vi "FleaRbRy.vi"() -> ()   [LabVIEW 2013]
doc: "Take a single PixelFly exposure and display the result as an intensity graph.This VI illustrates the basics of taking an exposure with the PixelFly camera. Use Ctrl-H to get help on any of the controls\n\nCopyright 2001, The Cooke Corporation."
uses:
  Shared Libraries/Controls/FileName_Cluster.ctl
  <vilib>/userdefined/High Color/IMAQdx.ctl
  <vilib>/vision/driver/IMAQdx.llb/IMAQdx Acquisition Mode.ctl
  <vilib>/addons/h5labview2/file/H5Fmode.ctl
  Shared Libraries/Controls/FileInfo_Global.vi
  <vilib>/addons/h5labview2/base/lib_path.vi
  <vilib>/addons/h5labview2/base/H5Equery.vi
  <vilib>/addons/h5labview2/base/hid_t.ctl
  <vilib>/addons/h5labview2/dataset/H5Dwrite.llb/H5Dwrite.xnode
  <vilib>/vision/driver/NI_Vision_Acquisition_Software.lvlib
  <vilib>/addons/h5labview2/file/H5F.lvlib
  <vilib>/addons/h5labview2/group/H5G.lvlib
panel:
  in  "Flea Acquire":bool=TRUE
  in  "Interrupt":bool
  out "Status":string="Running..."
  in  "stop":bool
  in  "Tab Control":enum32{"Setup", "Images", "Hardware status"}(tab)
  in  "Do Matlab Analysis":bool
  out "Matlab Command":string
  in  "Save Experimental Parameters to file":enum16{"False", "True"}(ring)
  in  "Flea File Parameters":T1={"Data Root"=path "C:/Data", "Index"=1, "Instrument"="FleaZ"} {"Index" format="%04d"}
  in  "Camera Name":T2="Flea3 FL3-GE-28S4M"
  in  "Experiment":T3(ring)=enum."RbRy"
  in  "Pull Setlist inform string":bool
  in  "Flea Magnification":dbl=1.0
  in  "Flea Image direction":enum16{"XY", "XZ", "ZAxis", "YAxis"}(ring)=enum."ZAxis"
  in  "Flea Imaging technique":enum16{"Absorption", "Fluorescence", "RawImage"}(ring)
  out "Image note":string="Experiment=Sr\nCamera_ID=Flea3_20S4M\nImageType=Raw\nDataType=Absorption\nImageDirection=XZ\nMagnification=6.630000E-1\nWMfreq=4.357345797E+2\nFileNumber=4534\nIndex=27\nIndexedWaves=BlueLaserLockOffset;DipPowX;DipPowX2;DipPowZ;DoppCoolDet;DoppCoolSweep;Nspacers;Pdet;ProbeDet;TOF;TOFaux;WMfreq;Xshim;Yshim;ZshimDC;ZshimVar;bLoadT;bMapT;combWidthF;combWidthI;depumpOn;depumpPow;dopCoolT;freq;holdT;loadT;rMOTbroadDetuningF;rMOTbroadDetuningI;rMOTon;rMOTpow2;rMOTpow3;rMOTpow4;rMOTpow5;rMOTstirDetF;rMOTstirDetI;singleFreqDet;singleFreqStirDet;varWaveP1\nIndexedValues=6.00000000000000E+0;3.00000000000000E+0;3.00000000000000E+0;2.00000000000000E+0;-1.36000000000000E+3;-20.0000000000000E+0;4.00000000000000E+0;4.25000000000000E+0;0.00000000000000E+0;15.0000000000000E-3;8.00000000000000E-3;0.00000000000000E+0;300.000000000000E-3;1.60000000000000E+0;1.65000000000000E+0;1.65000000000000E+0;9.90000000000000E+0;400.000000000000E-6;100.000000000000E-3;1.25000000000000E+0;1.00000000000000E+0;1.00000000000000E+0;75.0000000000000E-3;30.0000000000000E+3;400.000000000000E-3;35.0000000000000E-3;4.77500000000000E+0;4.40000000000000E+0;1.00000000000000E+0;3.00000000000000E+0;7.10000000000000E+0;4.00000000000000E+0;1.15000000000000E+0;4.50000000000000E+0;4.50000000000000E+0;-3.90000000000000E+3;-3.95000000000000E+3;3.50000000000000E+0\n# Current Variables\n#\ndepumpOn = 1.000000E+0\nBBcompT = 4.000000E-1\nBlueLaserLockOffset = 6.000000E+0\nDipPowX = 3.000000E+0\nDipPowX2 = 3.000000E+0\nDipPowXLat = 1.500000E+0\nDipPowZ = 2.000000E+0\nDipPowZ2 = 2.500000E-2\nDipPowZ3 = 2.500000E-2\nDoppCoolDet = -1.360000E+3\nDoppCoolSweep = -2.000000E+1\nHeatingAmp = 1.000000E+0\nMOTPow = 8.000000E+0\nMOTcurrent = -7.500000E+0\nMOTdetuning = -4.504000E+1\nNspacers = 4.000000E+0\nPdet = 4.250000E+0\nPdet2 = 5.000000E-2\nProbeDet = 0.000000E+0\nProbePow = 1.950000E+0\nTOF = 1.500000E-2\nTOFaux = 8.000000E-3\nWMfreq = 0.000000E+0\nXshim = 3.000000E-1\nXshimDC = 6.000000E-1\nYshim = 1.600000E+0\nYshimDC = 1.500000E+0\nZshim = 1.650000E+0\nZshimDC = 1.650000E+0\nZshimVar = 1.650000E+0\nbLoadT = 9.900000E+0\nbMapT = 4.000000E-4\ncombWidthF = 1.000000E-1\ncombWidthI = 1.250000E+0\ncompensation = -3.981000E+0\ndepumpPow = 1.000000E+0\ndopCoolT = 7.500000E-2\ndopCoolT1 = 5.000000E-3\nfreq = 3.000000E+4\nholdT = 4.000000E-1\nloadT = 3.500000E-2\nminus_zman = -7.904000E+0\nplus_zman = -9.792000E+0\nrMOTbroadDetuningF = 4.775000E+0\nrMOTbroadDetuningI = 4.400000E+0\nrMOTcurrF = -2.000000E-1\nrMOTcurrI = -2.000000E-1\nrMOTon = 1.000000E+0\nrMOTpow1 = 7.000000E+0\nrMOTpow2 = 3.000000E+0\nrMOTpow3 = 7.100000E+0\nrMOTpow4 = 4.000000E+0\nrMOTpow5 = 1.150000E+0\nrMOTpow6 = 0.000000E+0\nrMOTstirDetF = 4.500000E+0\nrMOTstirDetI = 4.500000E+0\nsingleFreqDet = -3.900000E+3\nsingleFreqStirDet = -3.950000E+3\nstirWidthF = 1.000000E-1\nstirWidthI = 1.250000E+0\ntEvap0 = 1.000000E-1\ntEvap1 = 2.000000E+0\ntEvap2 = 3.000000E-1\ntau = 6.000000E-1\nvarWaveP1 = 3.500000E+0\nvarWaveP2 = 3.500000E+0\n#\n# Master Staging List\n#Comment\tMarker\tMode\tGroup\tDelay\tX ODT Shuttter\tX ODT AO TTL\tY ODT Shutter\tY ODT AO TTL\tZ ODT Shutter\tZ ODT AO TTL\t707 Shutter\tPB_7\tPB_8\tFreq Switch rMOT\trMOT AO TTL\t\tTrans AO TTL\tProbe AO TTL\tZman AO TTL\tbMOT AO TTL\t60 Hz Trig Gate\tWindow Heater TTL\tPB_18\tPB_19\tPB_20 Trigger Dev3\tPB_21 Trigger Dev2\tPB_22 Trigger Dev1\tPB_23 Trigger Dev0\tStep\t~Atomic Beam Shutter\tGate Valve\tDO0_2\tDO0_3\t~Zman Coils\t~ MOT Coils\t~ Dipole Flea3 Shutter\trMOT Shutter\t+Zeeman Coils\t-Zeeman Coils\tCompensation Coils\tMOT Coils\trMOT AO Power\trMOT Freq Amplitude\trMOT Freq Offset\tAO0_7\tTrans Shutter\tProbe Shutter\tZman Shutter\tbMOT Shutter\tDO1_4\t679 Shutter\t~ Pixis Shutter\t~Abs Flea3 Shutter\tMOT AO Frequency\tMOT AO Power\tProbe AO Power\tProbe AO Frequency\tX Shim Coils\tY Shim Coils\tZ Shim Coils\tZ ODT AO Power\tPIXIS Ext Shutter\tD02_1\tD02_2\tD02_3\tD02_4\tD02_5\tD02_6\tD02_7\tAO2_0\tAO2_1\tD03_0\tD03_1\tD03_2\tD03_3\tD03_4\tD03_5\tD03_6\tD03_7\tAO3_0\tAO3_1\tAO3_2\tVariable Waveplate\t461 Spec Offset\tAO3_5\tAO3_6\tX ODT AO Power\tSRS Freq\tSRS Amp\tSRS Offset\tSRS Func Type\tRedMotDDS\tRedMotDDS_ 0\tRedMotDDS_ 1\tRedMotDDS_ 2\tStirringDDS\tStirringDDS_ 0\tStirringDDS_ 1\tStirringDDS_ 2\r\n\r\nreset\t\tRamp\t1\t.1\t1\t1\t0\t0\t1\t1\t1\t0\t0\t0\t1\t0\t1\t1\t1\t0\t0\t0\t0\t0\t0\t0\t0\t0\t0\t0\t1\t0\t1\t0\t0\t1\t0\tplus_zman\tminus_zman\tcompensation\tMOTcurrent\trMOTpow1\tcombAmplitude(combWidthI)\trMOTdelta(-(rMOTbroadDetuningI +combWidthI/2))\t0\t1\t0\t1\t1\t0\t1\t1\t1\tbMOTdelta(MOTdetuning)\tbMOTpow(0.5)\tProbePow\tPdet2\tXshim\tYshim\tZshim\tODTpowZ(DipPowZ)\t0\t0\t0\t0\t0\t0\t0\t0\t0\t0\t0\t0\t0\t0\t0\t0\t0\t0\trMOTdelta(-(rMOTstirDetI +stirWidthI/2))\tcombAmplitude(stirWidthI)\t0\tvarWaveP1\tBlueLaserLockOffset\tAmp688(depumpPow)\trMOTpow3\tODTpowX(DipPowX)\tfreq\tHeatingAmp\t0\tSine\tDetuning\tsingleFreqDet\t-20\t8\tDetuning\tsingleFreqStirDet\t0\t0\r\nblue MOT load\t\tRamp\t1\tbLoadT\t1\t1\t0\t0\t1\t1\t0\t0\t0\t0\t1\t0\t1\t1\t1\t1\t0\t0\t0\t0\t0\t0\t0\t0\t0\t0\t1\t0\t0\t0\t0\t1\t0\tplus_zman\tminus_zman\tcompensation\tMOTcurrent\trMOTpow1\tcombAmplitude(combWidthI)\trMOTdelta(-(rMOTbroadDetuningI +combWidthI/2))\t0\t1\t0\t1\t1\t0\t1\t1\t1\tbMOTdelta(MOTdetuning)\tbMOTpow(MOTPow)\tProbePow\tPdet2\tXshim\tYshim\tZshim\tODTpowZ(DipPowZ)\t0\tdepumpOn\t0\t0\t0\t0\t0\t0\t0\t0\t0\t0\t0\t0\t0\t0\t0\t0\trMOTdelta(-(rMOTstirDetI +stirWidthI/2))\tcombAmplitude(stirWidthI)\t0\tvarWaveP1\tBlueLaserLockOffset\tAmp688(depumpPow)\trMOTpow3\tODTpowX(DipPowX)\tfreq\tHeatingAmp\t0\tSine\tDetuning\tsingleFreqDet\t-20\t8\tDetuning\tsingleFreqStirDet\t0\t0\r\npretrig\t\tRamp\t1\t6.244e-3\t1\t1\t0\t0\t1\t1\t0\t0\t0\t0\t1\t0\t1\t1\t1\t1\t0\t1\t0\t0\t0\t0\t0\t0\t0\t0\t1\t0\t0\t0\t0\t0\t0\tplus_zman\tminus_zman\tcompensation\tMOTcurrent\trMOTpow1\tcombAmplitude(combWidthI)\trMOTdelta(-(rMOTbroadDetuningI +combWidthI/2))\t0\t1\t0\t1\t1\t0\t1\t0\t0\tbMOTdelta(MOTdetuning)\tbMOTpow(MOTPow)\tProbePow\tPdet2\tXshim\tYshim\tZshim\tODTpowZ(DipPowZ)\t0\tdepumpOn\t0\t0\t0\t0\t0\t0\t0\t0\t0\t0\t0\t0\t0\t0\t0\t0\trMOTdelta(-(rMOTstirDetI +stirWidthI/2))\tcombAmplitude(stirWidthI)\t0\tvarWaveP1\tBlueLaserLockOffset\tAmp688(depumpPow)\trMOTpow3\tODTpowX(DipPowX)\tfreq\tHeatingAmp\t0\tSine\tDetuning\tsingleFreqDet\t-20\t8\tDetuning\tsingleFreqStirDet\t0\t0\r\ndump bMOT\t\tRamp\t1\t0.1\t1\t1\t0\t0\t1\t1\t0\t0\t0\t0\t1\t0\t1\t1\t1\t1\t0\t1\t0\t0\t0\t0\t0\t0\t0\t0\t1\t0\t0\t0\t0\t1\t0\tplus_zman\tminus_zman\tcompensation\tMOTcurrent\trMOTpow1\tcombAmplitude(combWidthI)\trMOTdelta(-(rMOTbroadDetuningI +combWidthI/2))\t0\t1\t0\t1\t1\t0\t1\t1\t1\tbMOTdelta(MOTdetuning)\tbMOTpow(MOTPow)\tProbePow\tPdet2\tXshim\tYshim\tZshim\tODTpowZ(DipPowZ)\t0\tdepumpOn\t0\t0\t0\t0\t0\t0\t0\t0\t0\t0\t0\t0\t0\t0\t0\t0\trMOTdelta(-(rMOTstirDetI +stirWidthI/2))\tcombAmplitude(stirWidthI)\t0\tvarWaveP1\tBlueLaserLockOffset\tAmp688(depumpPow)\trMOTpow3\tODTpowX(DipPowX)\tfreq\tHeatingAmp\t0\tSine\tDetuning\tsingleFreqDet\t-20\t8\tDetuning\tsingleFreqStirDet\t0\t0\r\nCamWaitTime\t\tRamp\t1-rMOTon\t.1\t1\t1\t0\t0\t1\t1\t1\t0\t0\t0\t1\t0\t1\t0\t1\t1\t0\t1\t0\t0\t0\t0\t0\t0\t0\t0\t1\t0\t1\t0\t0\t1\t0\tplus_zman\tminus_zman\tcompensation\tMOTcurrent\trMOTpow1\tcombAmplitude(combWidthI)\trMOTdelta(-(rMOTbroadDetuningI +combWidthI/2))\t0\t1\t1\t1\t1\t0\t1\t1\t1\tbMOTdelta(MOTdetuning)\tbMOTpow(MOTPow)\tProbePow\tPdet2\tXshim\tYshim\tZshim\tODTpowZ(DipPowZ)\t0\t0\t0\t0\t0\t0\t0\t0\t0\t0\t0\t0\t0\t0\t0\t0\t0\t0\trMOTdelta(-(rMOTstirDetI +stirWidthI/2))\tcombAmplitude(stirWidthI)\t0\tvarWaveP1\tBlueLaserLockOffset\tAmp688(depumpPow)\trMOTpow3\tODTpowX(DipPowX)\tfreq\tHeatingAmp\t0\tSine\tDetuning\tsingleFreqDet\t-20\t8\tDetuning\tsingleFreqStirDet\t0\t0\r\nProbeShutOn\t\tRamp\t1-rMOTon\t1120e-6\t1\t1\t0\t0\t1\t1\t1\t0\t0\t0\t1\t0\t0\t0\t0\t1\t0\t1\t0\t0\t0\t0\t0\t0\t0\t0\t1\t0\t1\t0\t0\t1\t1\tplus_zman\tminus_zman\tcompensation\tMOTcurrent\trMOTpow1\tcombAmplitude(combWidthI)\trMOTdelta(-(rMOTbroadDetuningI +combWidthI/2))\t0\t1\t1\t1\t1\t0\t1\t1\t1\tbMOTdelta(MOTdetuning)\tbMOTpow(MOTPow)\tProbePow\tPdet2\tXshim\tYshim\tZshim\tODTpowZ(DipPowZ)\t0\t0\t0\t0\t0\t0\t0\t0\t0\t0\t0\t0\t0\t0\t0\t0\t0\t0\trMOTdelta(-(rMOTstirDetI +stirWidthI/2))\tcombAmplitude(stirWidthI)\t0\tvarWaveP1\tBlueLaserLockOffset\tAmp688(depumpPow)\trMOTpow3\tODTpowX(DipPowX)\tfreq\tHeatingAmp\t0\tSine\tDetuning\tsingleFreqDet\t-20\t8\tDetuning\tsingleFreqStirDet\t0\t0\r\nRepumpShutOff\t\tRamp\t1-rMOTon\t260e-6\t1\t1\t0\t0\t1\t1\t1\t0\t0\t0\t1\t0\t0\t0\t0\t1\t0\t1\t0\t0\t0\t0\t0\t0\t0\t0\t1\t0\t1\t0\t0\t1\t1\tplus_zman\tminus_zman\tcompensation\tMOTcurrent\trMOTpow1\tcombAmplitude(combWidthI)\trMOTdelta(-(rMOTbroadDetuningI +combWidthI/2))\t0\t1\t1\t0\t1\t0\t1\t1\t1\tbMOTdelta(MOTdetuning)\tbMOTpow(MOTPow)\tProbePow\tPdet2\tXshim\tYshim\tZshim\tODTpowZ(DipPowZ)\t0\t0\t0\t0\t0\t0\t0\t0\t0\t0\t0\t0\t0\t0\t0\t0\t0\t0\trMOTdelta(-(rMOTstirDetI +stirWidthI/2))\tcombAmplitude(stirWidthI)\t0\tvarWaveP1\tBlueLaserLockOffset\tAmp688(depumpPow)\trMOTpow3\tODTpowX(DipPowX)\tfreq\tHeatingAmp\t0\tSine\tDetuning\tsingleFreqDet\t-20\t8\tDetuning\tsingleFreqStirDet\t0\t0\r\nMOTShutOff\t\tRamp\t1-rMOTon\t1370e-6\t1\t1\t0\t0\t1\t1\t1\t0\t0\t0\t1\t0\t0\t0\t0\t1\t0\t1\t0\t0\t0\t0\t0\t0\t0\t0\t1\t0\t1\t0\t0\t1\t1\tplus_zman\tminus_zman\tcompensation\tMOTcurrent\trMOTpow1\tcombAmplitude(combWidthI)\trMOTdelta(-(rMOTbroadDetuningI +combWidthI/2))\t0\t1\t1\t0\t0\t0\t1\t1\t1\tbMOTdelta(MOTdetuning)\tbMOTpow(MOTPow)\tProbePow\tPdet2\tXshim\tYshim\tZshim\tODTpowZ(DipPowZ)\t0\t0\t0\t0\t0\t0\t0\t0\t0\t0\t0\t0\t0\t0\t0\t0\t0\t0\trMOTdelta(-(rMOTstirDetI +stirWidthI/2))\tcombAmplitude(stirWidthI)\t0\tvarWaveP1\tBlueLaserLockOffset\tAmp688(depumpPow)\trMOTpow3\tODTpowX(DipPowX)\tfreq\tHeatingAmp\t0\tSine\tDetuning\tsingleFreqDet\t-20\t8\tDetuning\tsingleFreqStirDet\t0\t0\r\nCoil Switch\t\tRamp\trMOTon\t220e-6\t1\t1\t0\t0\t1\t1\t1\t0\t0\t0\t1\t0\t0\t0\t0\t0\t0\t1\t0\t0\t0\t0\t0\t0\t0\t0\t1\t0\t1\t0\t0\t1\t1\tplus_zman\tminus_zman\tcompensation\trMOTcurrI\trMOTpow1\tcombAmplitude(combWidthI)\trMOTdelta(-(rMOTbroadDetuningI +combWidthI/2))\t0\t1\t1\t0\t0\t0\t1\t1\t1\tbMOTdelta(MOTdetuning)\tbMOTpow(0.5)\tProbePow\tPdet2\tXshim\tYshim\tZshim\tODTpowZ(DipPowZ)\t0\t0\t0\t0\t0\t0\t0\t0\t0\t0\t0\t0\t0\t0\t0\t0\t0\t0\trMOTdelta(-(rMOTstirDetI +stirWidthI/2))\tcombAmplitude(stirWidthI)\t0\tvarWaveP1\tBlueLaserLockOffset\tAmp688(depumpPow)\trMOTpow3\tODTpowX(DipPowX)\tfreq\tHeatingAmp\t0\tSine\tDetuning\tsingleFreqDet\t-20\t8\tDetuning\tsingleFreqStirDet\t0\t0\r\n60HzTrigger\t\tHalt\t0\t10u\t1\t1\t0\t0\t1\t1\t1\t0\t0\t0\t1\t0\t0\t0\t0\t0\t1\t1\t0\t0\t0\t0\t0\t0\t0\t0\t1\t0\t1\t0\t0\t1\t1\tplus_zman\tminus_zman\tcompensation\trMOTcurrI\trMOTpow1\tcombAmplitude(combWidthI)\trMOTdelta(-(rMOTbroadDetuningI +combWidthI/2))\t0\t1\t1\t0\t0\t0\t1\t1\t1\tbMOTdelta(MOTdetuning)\tbMOTpow(0.5)\tProbePow\tPdet2\tXshim\tYshim\tZshim\tODTpowZ(DipPowZ)\t0\t0\t0\t0\t0\t0\t0\t0\t0\t0\t0\t0\t0\t0\t0\t0\t0\t0\trMOTdelta(-(rMOTstirDetI +stirWidthI/2))\tcombAmplitude(stirWidthI)\t0\tvarWaveP1\tBlueLaserLockOffset\tAmp688(depumpPow)\trMOTpow3\tODTpowX(DipPowX)\tfreq\tHeatingAmp\t0\tSine\tDetuning\tsingleFreqDet\t-20\t8\tDetuning\tsingleFreqStirDet\t0\t0\r\nCapture Red MOT\t\tRamp\trMOTon\t.175\t1\t1\t0\t0\t1\t0\t1\t0\t0\t0\t1\t0\t0\t0\t0\t0\t0\t1\t0\t0\t0\t0\t0\t0\t0\t0\t1\t0\t1\t0\t0\t1\t1\tplus_zman\tminus_zman\tcompensation\trMOTcurrI\trMOTpow1\tcombAmplitude(combWidthI)\trMOTdelta(-(rMOTbroadDetuningI +combWidthI/2))\t0\t0\t0\t0\t0\t0\t1\t1\t1\tbMOTdelta(MOTdetuning)\tbMOTpow(0.5)\tProbePow\tPdet2\tXshim\tYshim\tZshim\tODTpowZ(DipPowZ)\t0\t0\t0\t0\t0\t0\t0\t0\t0\t0\t0\t0\t0\t0\t0\t0\t0\t0\trMOTdelta(-(rMOTstirDetI +stirWidthI/2))\tcombAmplitude(stirWidthI)\t0\tvarWaveP1\tBlueLaserLockOffset\tAmp688(depumpPow)\trMOTpow3\tODTpowX(DipPowX)\tfreq\tHeatingAmp\t0\tSine\tDetuning\tsingleFreqDet\t-20\t8\tDetuning\tsingleFreqStirDet\t0\t0\r\nRamp Red MOT\t\tRamp\t1\tBBcompT\t1\t1\t0\t0\t1\t0\t1\t0\t0\t0\t1\t0\t0\t0\t0\t0\t0\t1\t0\t0\t0\t0\t0\t0\t10u\t0\t1\t0\t1\t0\t0\t1\t1\tplus_zman\tminus_zman\tcompensation\tLineRamp(f,rMOTcurrI,rMOTcurrF)\tHalfGaussRamp(t,rMOTpow1,rMOTpow2, BBcompT)\tLineRamp(f,combAmplitude(combWidthI),combAmplitude(combWidthF))\tLineRamp(f,rMOTdelta(-(rMOTbroadDetuningI +combWidthI/2)),rMOTdelta(-(rMOTbroadDetuningF +combWidthF/2)))\t0\t0\t0\t0\t0\t0\t1\t0\t1\tbMOTdelta(MOTdetuning)\tbMOTpow(0.5)\tProbePow\tPdet2\tXshim\tYshim\tLineRamp(f,Zshim,ZshimVar)\tODTpowZ(DipPowZ)\t0\t0\t0\t0\t0\t0\t0\t0\t0\t0\t0\t0\t0\t0\t0\t0\t0\t0\tLineRamp(f,rMOTdelta(-(rMOTstirDetI +stirWidthI/2)),rMOTdelta(-(rMOTstirDetF +stirWidthF/2)))\tLineRamp(f,combAmplitude(stirWidthI),combAmplitude(stirWidthF))\t0\tvarWaveP1\tLineRamp(f,BlueLaserLockOffset,Pdet)\tAmp688(depumpPow)\tHalfGaussRamp(t,rMOTpow3,rMOTpow4, BBcompT)\tODTpowX(DipPowX)\tfreq\tHeatingAmp\t0\tSine\tDetuning\tsingleFreqDet\t-20\t8\tDetuning\tsingleFreqStirDet\t0\t0\r\nSF\t\tRamp\t0\t.025\t1\t1\t0\t0\t1\t0\t0\t0\t0\t1\t1\t0\t0\t0\t0\t0\t0\t1\t0\t0\t0\t0\t0\t0\t10u\t0\t1\t0\t0\t0\t0\t1\t1\tplus_zman\tminus_zman\tcompensation\trMOTcurrF\tLineRamp(f,rMOTpow2,rMOTpow2)\tcombAmplitude(combWidthF)\trMOTdelta(-(rMOTbroadDetuningF +combWidthF/2))\t0\t0\t0\t0\t0\t0\t0\t1\t1\tbMOTdelta(MOTdetuning)\tbMOTpow(0.5)\tProbePow\tPdet2\tXshim\tYshim\tZshimVar\tODTpowZ(DipPowZ)\t0\t0\t0\t0\t0\t0\t0\t0\t0\t0\t0\t0\t0\t0\t0\t0\t0\t0\trMOTdelta(-(rMOTstirDetI +stirWidthF/2))\tcombAmplitude(stirWidthF)\t0\tvarWaveP1\tPdet\tAmp688(depumpPow)\tLineRamp(f,rMOTpow4,rMOTpow4)\tODTpowX(DipPowX)\tfreq\tHeatingAmp\t0\tSine\tDetuning\tsingleFreqDet\t-20\t8\tDetuning\tsingleFreqStirDet\t0\t0\r\nload1\t\tRamp\t0\tloadT\t1\t1\t0\t0\t1\t0\t0\t0\t0\t1\t1\t0\t0\t1\t0\t0\t0\t1\t0\t0\t0\t0\t0\t0\t0\t0\t1\t0\t0\t0\t0\t1\t1\tplus_zman\tminus_zman\tcompensation\trMOTcurrF\trMOTpow3\tcombAmplitude(combWidthF)\trMOTdelta(-(rMOTbroadDetuningF +combWidthF/2))\t0\t0\t0\t0\t0\t0\t0\t1\t1\tbMOTdelta(MOTdetuning)\tbMOTpow(0.5)\tProbePow\tPdet2\tXshim\tYshim\tZshimVar\tODTpowZ(DipPowZ)\t0\t0\t0\t0\t0\t0\t0\t0\t0\t0\t0\t0\t0\t0\t0\t0\t0\t0\trMOTdelta(-(rMOTstirDetI +stirWidthF/2))\tcombAmplitude(stirWidthF)\t0\tvarWaveP1\tPdet\tAmp688(depumpPow)\trMOTpow3\tODTpowX(DipPowX)\tfreq\tHeatingAmp\t0\tSine\tDetuning\tsingleFreqDet\t-20\t8\tDetuning\tsingleFreqStirDet\t0\t0\r\nload2\t\tRamp\t0\t.05\t1\t1\t0\t0\t1\t0\t0\t0\t0\t1\t1\t0\t0\t1\t0\t0\t0\t1\t0\t0\t0\t0\t0\t0\t0\t0\t1\t0\t0\t0\t0\t1\t1\tplus_zman\tminus_zman\tcompensation\trMOTcurrF\trMOTpow3\tcombAmplitude(combWidthF)\trMOTdelta(-(rMOTbroadDetuningF +combWidthF/2))\t0\t0\t0\t0\t0\t0\t0\t1\t1\tbMOTdelta(MOTdetuning)\tbMOTpow(0.5)\tProbePow\tPdet2\tXshim\tYshim\tZshimVar\tODTpowZ(DipPowZ)\t0\t0\t0\t0\t0\t0\t0\t0\t0\t0\t0\t0\t0\t0\t0\t0\t0\t0\trMOTdelta(-(rMOTstirDetI +stirWidthF/2))\tcombAmplitude(stirWidthF)\t0\tvarWaveP1\tPdet\tAmp688(depumpPow)\trMOTpow3\tODTpowX(DipPowX)\tfreq\tHeatingAmp\t0\tSine\tDetuning\tsingleFreqDet\t-20\t8\tDetuning\tsingleFreqStirDet\t0\t0\r\ndrop Red MOT\t\tRamp\t0\t.05\t1\t1\t0\t0\t1\t0\t0\t0\t0\t1\t0\t0\t0\t1\t0\t0\t0\t1\t0\t0\t0\t0\t0\t0\t10u\t0\t1\t0\t0\t0\t1\t1\t0\tplus_zman\tminus_zman\tcompensation\trMOTcurrF\trMOTpow3\tcombAmplitude(combWidthF)\trMOTdelta(-(rMOTbroadDetuningF +combWidthF/2))\t0\t0\t0\t0\t0\t0\t0\t1\t1\tbMOTdelta(MOTdetuning)\tbMOTpow(0.5)\tProbePow\tPdet2\tLineRamp(f,Xshim,XshimDC)\tLineRamp(f,Yshim,YshimDC)\tLineRamp(f,ZshimVar,ZshimDC)\tODTpowZ(DipPowZ)\t0\t0\t0\t0\t0\t0\t0\t0\t0\t0\t0\t0\t0\t0\t0\t0\t0\t0\trMOTdelta(-(rMOTstirDetI +stirWidthF/2))\tcombAmplitude(stirWidthF)\t0\tvarWaveP1\tPdet\tAmp688(depumpPow)\trMOTpow3\tODTpowX(DipPowX)\tfreq\tHeatingAmp\t0\tSine\tDetuning\tsingleFreqDet\t-20\t8\tDetuning\tsingleFreqStirDet\t0\t0\r\nramp Trap\t\tRamp\t0\t.05\t1\t1\t0\t0\t1\t0\t0\t0\t0\t1\t0\t0\t0\t1\t0\t0\t0\t1\t0\t0\t0\t0\t0\t0\t10u\t0\t1\t0\t0\t0\t1\t1\t0\tplus_zman\tminus_zman\tcompensation\trMOTcurrF\trMOTpow3\tcombAmplitude(combWidthF)\trMOTdelta(-(rMOTbroadDetuningF +combWidthF/2))\t0\t0\t0\t0\t0\t0\t0\t1\t1\tbMOTdelta(MOTdetuning)\tbMOTpow(0.5)\tProbePow\tPdet2\tXshimDC\tYshimDC\tZshimDC\tODTpowZ(DipPowZ)\t0\t0\t0\t0\t0\t0\t0\t0\t0\t0\t0\t0\t0\t0\t0\t0\t0\t0\trMOTdelta(-(rMOTstirDetI +stirWidthF/2))\tcombAmplitude(stirWidthF)\t0\tvarWaveP1\tPdet\tAmp688(depumpPow)\trMOTpow3\tSinRamp(t,(ODTpowX(DipPowX)+ODTpowX(DipPowX2))/2,(ODTpowX(DipPowX2)-ODTpowX(DipPowX))/2,10,3*pi/2)\tfreq\tHeatingAmp\t0\tSine\tDetuning\tsingleFreqDet\t-20\t8\tDetuning\tsingleFreqStirDet\t0\t0\r\nhold\t\tRamp\t0\t5\t1\t1\t0\t0\t1\t0\t0\t0\t0\t1\t0\t0\t0\t1\t0\t0\t0\t1\t0\t0\t0\t0\t0\t0\t0\t0\t1\t0\t0\t0\t1\t1\t1\tplus_zman\tminus_zman\tcompensation\trMOTcurrF\trMOTpow4\tcombAmplitude(combWidthF)\trMOTdelta(-(rMOTbroadDetuningF +combWidthF/2))\t0\t0\t0\t0\t0\t0\t0\t1\t1\tbMOTdelta(MOTdetuning)\tbMOTpow(0.5)\tProbePow\tPdet2\tXshimDC\tYshimDC\tZshimDC\tODTpowZ(DipPowZ)\t0\t0\t0\t0\t0\t0\t0\t0\t0\t0\t0\t0\t0\t0\t0\t0\t0\t0\trMOTdelta(-(rMOTstirDetI +stirWidthF/2))\tcombAmplitude(stirWidthF)\t0\tvarWaveP1\tPdet\tAmp688(depumpPow)\trMOTpow4\tODTpowX(DipPowX2)\tfreq\tHeatingAmp\t0\tSine\tDetuning\tDoppCoolDet\t-20\t8\tDetuning\tsingleFreqStirDet\t0\t0\r\nDoppler Cool1\t\tRamp\t0\tdopCoolT\t1\t1\t0\t0\t1\t0\t0\t0\t0\t1\t1\t0\t0\t1\t0\t0\t0\t1\t0\t0\t0\t0\t0\t0\t10u\t0\t1\t0\t0\t0\t1\t1\t1\tplus_zman\tminus_zman\tcompensation\trMOTcurrF\tLineRamp(f,rMOTpow4,1.15)\tcombAmplitude(combWidthF)\trMOTdelta(-(rMOTbroadDetuningF +combWidthF/2))\t0\t0\t0\t0\t0\t0\t0\t1\t1\tbMOTdelta(MOTdetuning)\tbMOTpow(0.5)\tProbePow\tPdet2\tXshimDC\tYshimDC\tZshimDC\tODTpowZ(DipPowZ)\t0\t0\t0\t0\t0\t0\t0\t0\t0\t0\t0\t0\t0\t0\t0\t0\t0\t0\trMOTdelta(-(rMOTstirDetI +stirWidthF/2))\tcombAmplitude(stirWidthF)\t0\tvarWaveP1\tPdet\tAmp688(depumpPow)\tLineRamp(f,rMOTpow4,1.15)\tODTpowX(DipPowX2)\tfreq\tHeatingAmp\t0\tSine\tDetuning\tDoppCoolDet\t-20\t8\tDetuning\tsingleFreqStirDet\t0\t0\r\nDoppler Cool2\t\tRamp\t0\tdopCoolT\t1\t1\t0\t0\t1\t0\t0\t0\t0\t1\t1\t0\t0\t1\t0\t0\t0\t1\t0\t0\t0\t0\t0\t0\t10u\t0\t1\t0\t0\t0\t1\t1\t1\tplus_zman\tminus_zman\tcompensation\trMOTcurrF\trMOTpow4\tcombAmplitude(combWidthF)\trMOTdelta(-(rMOTbroadDetuningF +combWidthF/2))\t0\t0\t0\t0\t0\t0\t0\t1\t1\tbMOTdelta(MOTdetuning)\tbMOTpow(0.5)\tProbePow\tPdet2\tXshimDC\tYshimDC\tZshimDC\tODTpowZ(DipPowZ)\t0\t0\t0\t0\t0\t0\t0\t0\t0\t0\t0\t0\t0\t0\t0\t0\t0\t0\trMOTdelta(-(rMOTstirDetI +stirWidthF/2))\tcombAmplitude(stirWidthF)\t0\tvarWaveP1\tPdet\tAmp688(depumpPow)\trMOTpow4\tODTpowX(DipPowX2)\tfreq\tHeatingAmp\t0\tSine\tRamp\tDoppCoolDet\tDoppCoolDet-DoppCoolSweep\tdopCoolT*1000\tDetuning\tsingleFreqStirDet\t0\t0\r\nDoppler Cool3\t\tRamp\t0\tdopCoolT\t1\t1\t0\t0\t1\t0\t0\t0\t0\t1\t1\t0\t0\t1\t0\t0\t0\t1\t0\t0\t0\t0\t0\t0\t10u\t0\t1\t0\t0\t0\t1\t1\t1\tplus_zman\tminus_zman\tcompensation\trMOTcurrF\tLineRamp(f,rMOTpow4,rMOTpow5)\tcombAmplitude(combWidthF)\trMOTdelta(-(rMOTbroadDetuningF +combWidthF/2))\t0\t0\t0\t0\t0\t0\t0\t1\t1\tbMOTdelta(MOTdetuning)\tbMOTpow(0.5)\tProbePow\tPdet2\tXshimDC\tYshimDC\tZshimDC\tODTpowZ(DipPowZ)\t0\t0\t0\t0\t0\t0\t0\t0\t0\t0\t0\t0\t0\t0\t0\t0\t0\t0\trMOTdelta(-(rMOTstirDetI +stirWidthF/2))\tcombAmplitude(stirWidthF)\t0\tvarWaveP1\tPdet\tAmp688(depumpPow)\tLineRamp(f,rMOTpow4,rMOTpow5)\tODTpowX(DipPowX2)\tfreq\tHeatingAmp\t0\tSine\tDetuning\tDoppCoolDet-DoppCoolSweep\tDoppCoolDet-DoppCoolSweep\tdopCoolT*1000\tDetuning\tsingleFreqStirDet\t0\t0\r\nhold\t\tRamp\t0\tholdT\t1\t1\t0\t0\t1\t0\t0\t0\t0\t1\t0\t0\t0\t1\t0\t0\t0\t1\t1\t0\t0\t0\t0\t0\t0\t0\t1\t0\t0\t0\t1\t1\t0\tplus_zman\tminus_zman\tcompensation\trMOTcurrF\trMOTpow4\tcombAmplitude(combWidthF)\trMOTdelta(-(rMOTbroadDetuningF +combWidthF/2))\t0\t1\t0\t0\t0\t0\t0\t1\t1\tbMOTdelta(MOTdetuning)\tbMOTpow(0.5)\tProbePow\tPdet2\tXshim\tYshim\tZshimVar\tODTpowZ(DipPowZ)\t0\t0\t0\t0\t0\t0\t0\t0\t0\t0\t0\t0\t0\t0\t0\t0\t0\t0\trMOTdelta(-(rMOTstirDetI +stirWidthF/2))\tcombAmplitude(stirWidthF)\t0\tvarWaveP1\tPdet\tAmp688(depumpPow)\trMOTpow4\tODTpowX(DipPowX2)\tfreq\tHeatingAmp\t0\tSine\tDetuning\tDoppCoolDet-DoppCoolSweep\tDoppCoolDet-DoppCoolSweep\tdopCoolT*1000\tDetuning\tsingleFreqStirDet\t0\t0\r\ndrop HTrap\t\tRamp\t0\t.03\t1\t1\t0\t0\t1\t0\t1\t0\t0\t1\t0\t0\t0\t1\t0\t0\t0\t1\t0\t0\t0\t0\t0\t0\t0\t0\t1\t0\t0\t0\t0\t1\t0\tplus_zman\tminus_zman\tcompensation\trMOTcurrF\trMOTpow3\tcombAmplitude(combWidthF)\trMOTdelta(-(rMOTbroadDetuningF +combWidthF/2))\t0\t1\t0\t0\t0\t0\t1\t1\t1\tbMOTdelta(MOTdetuning)\tbMOTpow(0.5)\tProbePow\tPdet2\tXshim\tYshim\tZshimVar\tODTpowZ(DipPowZ)\t0\t0\t0\t0\t0\t0\t0\t0\t0\t0\t0\t0\t0\t0\t0\t0\t0\t0\trMOTdelta(-(rMOTstirDetI +stirWidthF/2))\tcombAmplitude(stirWidthF)\t0\tvarWaveP1\tPdet\tAmp688(depumpPow)\trMOTpow3\tODTpowX(DipPowX)\tfreq\tHeatingAmp\t0\tSine\tDetuning\tsingleFreqDet\tDoppCoolDet-DoppCoolSweep\tdopCoolT*1000\tDetuning\tsingleFreqStirDet\t0\t0\r\nmodulate\t\tRamp\t0\t3m\t1\t1\t0\t0\t1\t0\t1\t0\t0\t1\t0\t0\t0\t1\t0\t0\t0\t1\t0\t0\t0\t0\t0\t0\t0\t0\t1\t0\t0\t0\t0\t1\t0\tplus_zman\tminus_zman\tcompensation\trMOTcurrF\trMOTpow3\tcombAmplitude(combWidthF)\trMOTdelta(-(rMOTbroadDetuningF +combWidthF/2))\t0\t1\t0\t0\t0\t0\t1\t1\t1\tbMOTdelta(MOTdetuning)\tbMOTpow(0.5)\tProbePow\tPdet2\tXshim\tYshim\tZshimVar\tODTpowZ(DipPowZ)\t0\t0\t0\t0\t0\t0\t0\t0\t0\t0\t0\t0\t0\t0\t0\t0\t0\t0\trMOTdelta(-(rMOTstirDetI +stirWidthF/2))\tcombAmplitude(stirWidthF)\t0\tvarWaveP1\tPdet\tAmp688(depumpPow)\trMOTpow3\tODTpowX(DipPowX)\tfreq\tHeatingAmp\t0\tSine\tDetuning\tsingleFreqDet\tDoppCoolDet-DoppCoolSweep\tdopCoolT*1000\tDetuning\tsingleFreqStirDet\t0\t0\r\nEvaporation\t\tRamp\t0\ttEvap1\t1\t1\t0\t0\t1\t0\t1\t0\t0\t1\t0\t0\t0\t1\t0\t0\t0\t1\t0\t0\t0\t0\t0\t0\t1m\t0\t1\t0\t0\t0\t0\t1\t0\tplus_zman\tminus_zman\tcompensation\trMOTcurrF\trMOTpow3\tcombAmplitude(combWidthF)\trMOTdelta(-(rMOTbroadDetuningF +combWidthF/2))\t0\t1\t0\t0\t0\t0\t1\t1\t1\tbMOTdelta(MOTdetuning)\tbMOTpow(0.5)\tProbePow\tPdet2\tXshim\tYshim\tZshimVar\tODTpowZ(DipPowZ)\t0\t0\t0\t0\t0\t0\t0\t0\t0\t0\t0\t0\t0\t0\t0\t0\t0\t0\trMOTdelta(-(rMOTstirDetI +stirWidthF/2))\tcombAmplitude(stirWidthF)\t0\tvarWaveP1\tPdet\tAmp688(depumpPow)\trMOTpow3\tExpRamp2(t,0,ODTpowX(DipPowX),ODTpowX(DipPowX2),tau)\tfreq\tHeatingAmp\t0\tSine\tDetuning\tsingleFreqDet\tDoppCoolDet-DoppCoolSweep\tdopCoolT*1000\tDetuning\tsingleFreqStirDet\t0\t0\r\ndrop\t\tRamp\t0\t.01\t1\t1\t0\t0\t1\t0\t1\t0\t0\t1\t0\t0\t0\t1\t0\t0\t0\t1\t0\t0\t0\t0\t0\t0\t0\t0\t1\t0\t0\t0\t0\t1\t0\tplus_zman\tminus_zman\tcompensation\trMOTcurrF\trMOTpow3\tcombAmplitude(combWidthF)\trMOTdelta(-(rMOTbroadDetuningF +combWidthF/2))\t0\t1\t0\t0\t0\t0\t1\t1\t1\tbMOTdelta(MOTdetuning)\tbMOTpow(0.5)\tProbePow\tPdet2\tXshim\tYshim\tZshimVar\tODTpowZ(DipPowZ)\t0\t0\t0\t0\t0\t0\t0\t0\t0\t0\t0\t0\t0\t0\t0\t0\t0\t0\trMOTdelta(-(rMOTstirDetI +stirWidthF/2))\tcombAmplitude(stirWidthF)\t0\tvarWaveP2\tPdet\tAmp688(depumpPow)\trMOTpow3\tODTpowX(DipPowXLat)\tfreq\tHeatingAmp\t0\tSine\tDetuning\tsingleFreqDet\tDoppCoolDet-DoppCoolSweep\tdopCoolT*1000\tDetuning\tsingleFreqStirDet\t0\t0\r\nband map\t\tRamp\t0\tbMapT\t1\t1\t0\t0\t1\t0\t1\t0\t0\t1\t0\t0\t0\t1\t0\t0\t0\t1\t0\t0\t0\t0\t0\t0\t2u\t0\t1\t0\t0\t0\t0\t1\t0\tplus_zman\tminus_zman\tcompensation\trMOTcurrF\trMOTpow3\tcombAmplitude(combWidthF)\trMOTdelta(-(rMOTbroadDetuningF +combWidthF/2))\t0\t1\t0\t0\t0\t0\t1\t1\t1\tbMOTdelta(MOTdetuning)\tbMOTpow(0.5)\tProbePow\tPdet2\tXshim\tYshim\tZshimVar\tLineRamp(f,ODTpowZ(DipPowZ),ODTpowZ(-0.2))\t0\t0\t0\t0\t0\t0\t0\t0\t0\t0\t0\t0\t0\t0\t0\t0\t0\t0\trMOTdelta(-(rMOTstirDetI +stirWidthF/2))\tcombAmplitude(stirWidthF)\t0\tvarWaveP2\tPdet\tAmp688(depumpPow)\trMOTpow3\tLineRamp(f,ODTpowX(DipPowX),0)\tfreq\tHeatingAmp\t0\tSine\tDetuning\tsingleFreqDet\tDoppCoolDet-DoppCoolSweep\tdopCoolT*1000\tDetuning\tsingleFreqStirDet\t0\t0\r\nband map delay\t\tRamp\t0\t10u\t1\t1\t0\t0\t1\t0\t1\t0\t0\t1\t0\t0\t0\t1\t0\t0\t0\t1\t0\t0\t0\t0\t0\t0\t0\t0\t1\t0\t0\t0\t0\t1\t0\tplus_zman\tminus_zman\tcompensation\trMOTcurrF\trMOTpow3\tcombAmplitude(combWidthF)\trMOTdelta(-(rMOTbroadDetuningF +combWidthF/2))\t0\t1\t0\t0\t0\t0\t1\t1\t1\tbMOTdelta(MOTdetuning)\tbMOTpow(0.5)\tProbePow\tPdet2\tXshim\tYshim\tZshimVar\tODTpowZ(DipPowZ)\t0\t0\t0\t0\t0\t0\t0\t0\t0\t0\t0\t0\t0\t0\t0\t0\t0\t0\trMOTdelta(-(rMOTstirDetI +stirWidthF/2))\tcombAmplitude(stirWidthF)\t0\tvarWaveP2\tPdet\tAmp688(depumpPow)\trMOTpow3\tODTpowX(DipPowXLat)\tfreq\tHeatingAmp\t0\tSine\tDetuning\tsingleFreqDet\tDoppCoolDet-DoppCoolSweep\tdopCoolT*1000\tDetuning\tsingleFreqStirDet\t0\t0\r\nTOF\t\tRamp\t0\tTOFaux\t0\t0\t0\t0\t0\t0\t1\t0\t0\t0\t0\t0\t0\t0\t0\t0\t0\t1\t0\t0\t0\t0\t0\t0\t0\t0\t1\t0\t0\t0\t1\t1\t0\tplus_zman\tminus_zman\tcompensation\trMOTcurrF\trMOTpow3\tcombAmplitude(combWidthF)\trMOTdelta(-(rMOTbroadDetuningF +combWidthF/2))\t0\t1\t1\t0\t0\t0\t1\t1\t1\tbMOTdelta(MOTdetuning)\tbMOTpow(0.5)\tProbePow\tPdet\tXshim\tYshim\tZshimVar\tODTpowZ(DipPowZ)\t1\t0\t0\t0\t0\t0\t0\t0\t0\t0\t0\t0\t0\t0\t0\t0\t0\t0\trMOTdelta(-(rMOTstirDetI +stirWidthF/2))\tcombAmplitude(stirWidthF)\t0\tvarWaveP2\tPdet\tAmp688(depumpPow)\trMOTpow3\tODTpowX(DipPowX2)\tfreq\tHeatingAmp\t0\tSine\tDetuning\tsingleFreqDet\tDoppCoolDet-DoppCoolSweep\tdopCoolT*1000\tDetuning\tsingleFreqStirDet\t0\t0\r\nTOF\t\tRamp\trMOTon\t.005\t0\t0\t0\t0\t0\t0\t1\t0\t0\t0\t0\t0\t0\t0\t0\t0\t0\t1\t0\t0\t0\t0\t0\t0\t0\t0\t1\t0\t0\t0\t1\t1\t0\tplus_zman\tminus_zman\tcompensation\trMOTcurrF\trMOTpow3\tcombAmplitude(combWidthF)\trMOTdelta(-(rMOTbroadDetuningF +combWidthF/2))\t0\t1\t1\t0\t0\t0\t1\t1\t1\tbMOTdelta(MOTdetuning)\tbMOTpow(0.5)\tProbePow\tPdet\tXshim\tYshim\tZshimVar\tODTpowZ(DipPowZ)\t1\t0\t0\t0\t0\t0\t0\t0\t0\t0\t0\t0\t0\t0\t0\t0\t0\t0\trMOTdelta(-(rMOTstirDetI +stirWidthF/2))\tcombAmplitude(stirWidthF)\t0\tvarWaveP2\tPdet\tAmp688(depumpPow)\trMOTpow3\tODTpowX(DipPowX2)\tfreq\tHeatingAmp\t0\tSine\tDetuning\tsingleFreqDet\tDoppCoolDet-DoppCoolSweep\tdopCoolT*1000\tDetuning\tsingleFreqStirDet\t0\t0\r\nTOF\t\tRamp\t1-rMOTon\t.001\t0\t0\t0\t0\t0\t0\t1\t0\t0\t0\t0\t0\t0\t0\t0\t0\t0\t1\t0\t0\t0\t0\t0\t0\t0\t0\t1\t0\t0\t0\t1\t1\t0\tplus_zman\tminus_zman\tcompensation\trMOTcurrF\trMOTpow3\tcombAmplitude(combWidthF)\trMOTdelta(-(rMOTbroadDetuningF +combWidthF/2))\t0\t1\t1\t0\t0\t0\t1\t1\t1\tbMOTdelta(MOTdetuning)\tbMOTpow(0.5)\tProbePow\tPdet\tXshim\tYshim\tZshimVar\tODTpowZ(DipPowZ)\t1\t0\t0\t0\t0\t0\t0\t0\t0\t0\t0\t0\t0\t0\t0\t0\t0\t0\trMOTdelta(-(rMOTstirDetI +stirWidthF/2))\tcombAmplitude(stirWidthF)\t0\tvarWaveP2\tPdet\tAmp688(depumpPow)\trMOTpow3\tODTpowX(DipPowX2)\tfreq\tHeatingAmp\t0\tSine\tDetuning\tsingleFreqDet\tDoppCoolDet-DoppCoolSweep\tdopCoolT*1000\tDetuning\tsingleFreqStirDet\t0\t0\r\narm FLEA\t\tRamp\t1\t.000044\t0\t0\t0\t0\t0\t0\t1\t0\t0\t0\t0\t0\t0\t0\t0\t0\t0\t0\t0\t0\t0\t0\t0\t0\t0\t0\t1\t0\t0\t0\t1\t0\t0\tplus_zman\tminus_zman\tcompensation\trMOTcurrF\trMOTpow3\tcombAmplitude(combWidthF)\trMOTdelta(-(rMOTbroadDetuningF +combWidthF/2))\t0\t1\t1\t0\t0\t0\t1\t1\t0\tbMOTdelta(MOTdetuning)\tbMOTpow(0.5)\tProbePow\tPdet\tXshim\tYshim\tZshimVar\tODTpowZ(0)\t1\t0\t0\t0\t0\t0\t0\t0\t0\t0\t0\t0\t0\t0\t0\t0\t0\t0\trMOTdelta(-(rMOTstirDetI +stirWidthF/2))\tcombAmplitude(stirWidthF)\t0\tvarWaveP2\tPdet\tAmp688(depumpPow)\trMOTpow3\tODTpowX(DipPowX)\tfreq\tHeatingAmp\t0\tSine\tDetuning\tsingleFreqDet\tDoppCoolDet-DoppCoolSweep\tdopCoolT*1000\tDetuning\tsingleFreqStirDet\t0\t0\r\natom img\t\tRamp\t1\t10e-6\t0\t0\t0\t0\t0\t0\t1\t0\t0\t0\t0\t0\t0\t1\t0\t0\t0\t0\t0\t0\t0\t0\t0\t0\t0\t0\t1\t0\t0\t0\t1\t0\t0\tplus_zman\tminus_zman\tcompensation\trMOTcurrF\trMOTpow3\tcombAmplitude(combWidthF)\trMOTdelta(-(rMOTbroadDetuningF +combWidthF/2))\t0\t1\t1\t0\t0\t0\t1\t0\t0\tbMOTdelta(MOTdetuning)\tbMOTpow(0.5)\tProbePow\tPdet\tXshim\tYshim\tZshimVar\tODTpowZ(0)\t1\t0\t0\t0\t0\t0\t0\t0\t0\t0\t0\t0\t0\t0\t0\t0\t0\t0\trMOTdelta(-(rMOTstirDetI +stirWidthF/2))\tcombAmplitude(stirWidthF)\t0\tvarWaveP2\tPdet\tAmp688(depumpPow)\trMOTpow3\tODTpowX(DipPowX)\tfreq\tHeatingAmp\t0\tSine\tDetuning\tsingleFreqDet\tDoppCoolDet-DoppCoolSweep\tdopCoolT*1000\tDetuning\tsingleFreqStirDet\t0\t0\r\natom img\t\tRamp\t0\t2.8e-3\t0\t0\t0\t0\t0\t0\t1\t0\t0\t1\t0\t0\t0\t0\t0\t0\t0\t0\t0\t0\t0\t0\t0\t0\t0\t0\t1\t0\t0\t0\t1\t1\t0\tplus_zman\tminus_zman\tcompensation\trMOTcurrF\trMOTpow3\tcombAmplitude(combWidthF)\trMOTdelta(-(rMOTbroadDetuningF +combWidthF/2))\t0\t1\t1\t0\t0\t0\t1\t1\t1\tbMOTdelta(MOTdetuning)\tbMOTpow(0.5)\tProbePow\tPdet\tXshim\tYshim\tZshimVar\tODTpowZ(DipPowZ)\t1\t0\t0\t0\t0\t0\t0\t0\t0\t0\t0\t0\t0\t0\t0\t0\t0\t0\trMOTdelta(-(rMOTstirDetI +stirWidthF/2))\tcombAmplitude(stirWidthF)\t0\tvarWaveP2\tPdet\tAmp688(depumpPow)\trMOTpow3\tODTpowX(DipPowX)\tfreq\tHeatingAmp\t0\tSine\tDetuning\tsingleFreqDet\tDoppCoolDet-DoppCoolSweep\tdopCoolT*1000\tDetuning\tsingleFreqStirDet\t0\t0\r\ntransmit img\t\tRamp\t1\t.300\t0\t0\t0\t0\t0\t0\t1\t0\t0\t1\t0\t0\t0\t0\t0\t0\t0\t0\t0\t0\t0\t0\t0\t0\t0\t0\t1\t0\t0\t0\t1\t1\t0\tplus_zman\tminus_zman\tcompensation\trMOTcurrF\trMOTpow3\tcombAmplitude(combWidthF)\trMOTdelta(-(rMOTbroadDetuningF +combWidthF/2))\t0\t1\t1\t0\t0\t0\t1\t1\t1\tbMOTdelta(MOTdetuning)\tbMOTpow(0.5)\tProbePow\tPdet\tXshim\tYshim\tZshimVar\tODTpowZ(DipPowZ)\t1\t0\t0\t0\t0\t0\t0\t0\t0\t0\t0\t0\t0\t0\t0\t0\t0\t0\trMOTdelta(-(rMOTstirDetI +stirWidthF/2))\tcombAmplitude(stirWidthF)\t0\tvarWaveP2\tPdet\tAmp688(depumpPow)\trMOTpow3\tODTpowX(DipPowX)\tfreq\tHeatingAmp\t0\tSine\tDetuning\tsingleFreqDet\tDoppCoolDet-DoppCoolSweep\tdopCoolT*1000\tDetuning\tsingleFreqStirDet\t0\t0\r\narm PIXIS\t\tRamp\t1\t.007\t1\t1\t0\t0\t0\t1\t1\t0\t0\t1\t1\t0\t0\t0\t1\t1\t0\t0\t0\t0\t0\t0\t0\t0\t0\t0\t1\t0\t0\t0\t1\t1\t0\tplus_zman\tminus_zman\tcompensation\trMOTcurrF\trMOTpow1\tcombAmplitude(combWidthF)\trMOTdelta(-(rMOTbroadDetuningF +combWidthF/2))\t0\t1\t1\t0\t0\t0\t1\t1\t1\tbMOTdelta(MOTdetuning)\tbMOTpow(0.5)\tProbePow\tPdet\tXshim\tYshim\tZshimVar\tODTpowZ(DipPowZ)\t1\t0\t0\t0\t0\t0\t0\t0\t0\t0\t0\t0\t0\t0\t0\t0\t0\t0\trMOTdelta(-(rMOTstirDetI +stirWidthF/2))\tcombAmplitude(stirWidthF)\t0\tvarWaveP2\tPdet\tAmp688(depumpPow)\trMOTpow1\tODTpowX(DipPowX)\tfreq\tHeatingAmp\t0\tSine\tDetuning\tsingleFreqDet\tDoppCoolDet-DoppCoolSweep\tdopCoolT*1000\tDetuning\tsingleFreqStirDet\t0\t0\r\narm FLEA\t\tRamp\t1\t44e-6\t1\t1\t0\t0\t0\t1\t1\t0\t0\t1\t1\t0\t0\t0\t1\t1\t0\t0\t0\t0\t0\t0\t0\t0\t0\t0\t1\t0\t0\t0\t1\t0\t0\tplus_zman\tminus_zman\tcompensation\trMOTcurrF\trMOTpow1\tcombAmplitude(combWidthF)\trMOTdelta(-(rMOTbroadDetuningF +combWidthF/2))\t0\t1\t1\t0\t0\t0\t1\t1\t0\tbMOTdelta(MOTdetuning)\tbMOTpow(0.5)\tProbePow\tPdet\tXshim\tYshim\tZshimVar\tODTpowZ(DipPowZ)\t1\t0\t0\t0\t0\t0\t0\t0\t0\t0\t0\t0\t0\t0\t0\t0\t0\t0\trMOTdelta(-(rMOTstirDetI +stirWidthF/2))\tcombAmplitude(stirWidthF)\t0\tvarWaveP2\tPdet\tAmp688(depumpPow)\trMOTpow1\tODTpowX(DipPowX)\tfreq\tHeatingAmp\t0\tSine\tDetuning\tsingleFreqDet\tDoppCoolDet-DoppCoolSweep\tdopCoolT*1000\tDetuning\tsingleFreqStirDet\t0\t0\r\nprobe img\t\tRamp\t1\t10e-6\t1\t1\t0\t0\t0\t1\t1\t0\t0\t1\t1\t0\t0\t1\t1\t1\t0\t0\t0\t0\t0\t0\t0\t0\t0\t0\t1\t0\t0\t0\t1\t0\t0\tplus_zman\tminus_zman\tcompensation\trMOTcurrF\trMOTpow1\tcombAmplitude(combWidthF)\trMOTdelta(-(rMOTbroadDetuningF +combWidthF/2))\t0\t1\t1\t0\t0\t0\t1\t0\t0\tbMOTdelta(MOTdetuning)\tbMOTpow(0.5)\tProbePow\tPdet\tXshim\tYshim\tZshimVar\tODTpowZ(DipPowZ)\t1\t0\t0\t0\t0\t0\t0\t0\t0\t0\t0\t0\t0\t0\t0\t0\t0\t0\trMOTdelta(-(rMOTstirDetI +stirWidthF/2))\tcombAmplitude(stirWidthF)\t0\tvarWaveP2\tPdet\tAmp688(depumpPow)\trMOTpow1\tODTpowX(DipPowX)\tfreq\tHeatingAmp\t0\tSine\tDetuning\tsingleFreqDet\tDoppCoolDet-DoppCoolSweep\tdopCoolT*1000\tDetuning\tsingleFreqStirDet\t0\t0\r\nprobe img\t\tRamp\t0\t2.8e-3\t1\t1\t0\t0\t0\t1\t1\t0\t0\t1\t1\t0\t0\t0\t1\t1\t0\t0\t0\t0\t0\t0\t0\t0\t0\t0\t1\t0\t0\t0\t1\t1\t0\tplus_zman\tminus_zman\tcompensation\trMOTcurrF\trMOTpow1\tcombAmplitude(combWidthF)\trMOTdelta(-(rMOTbroadDetuningF +combWidthF/2))\t0\t1\t1\t0\t0\t0\t1\t1\t1\tbMOTdelta(MOTdetuning)\tbMOTpow(0.5)\tProbePow\tPdet\tXshim\tYshim\tZshimVar\tODTpowZ(DipPowZ)\t1\t0\t0\t0\t0\t0\t0\t0\t0\t0\t0\t0\t0\t0\t0\t0\t0\t0\trMOTdelta(-(rMOTstirDetI +stirWidthF/2))\tcombAmplitude(stirWidthF)\t0\tvarWaveP2\tPdet\tAmp688(depumpPow)\trMOTpow1\tODTpowX(DipPowX)\tfreq\tHeatingAmp\t0\tSine\tDetuning\tsingleFreqDet\tDoppCoolDet-DoppCoolSweep\tdopCoolT*1000\tDetuning\tsingleFreqStirDet\t0\t0\r\ntransmit img\t\tRamp\t1\t.3\t1\t1\t0\t0\t0\t1\t1\t0\t0\t1\t1\t0\t0\t0\t1\t1\t0\t0\t0\t0\t0\t0\t0\t0\t0\t0\t1\t0\t0\t0\t1\t1\t0\tplus_zman\tminus_zman\tcompensation\trMOTcurrF\trMOTpow1\tcombAmplitude(combWidthF)\trMOTdelta(-(rMOTbroadDetuningF +combWidthF/2))\t0\t1\t1\t0\t0\t0\t1\t1\t1\tbMOTdelta(MOTdetuning)\tbMOTpow(0.5)\tProbePow\tPdet\tXshim\tYshim\tZshimVar\tODTpowZ(DipPowZ)\t1\t0\t0\t0\t0\t0\t0\t0\t0\t0\t0\t0\t0\t0\t0\t0\t0\t0\trMOTdelta(-(rMOTstirDetI +stirWidthF/2))\tcombAmplitude(stirWidthF)\t0\tvarWaveP2\tPdet\tAmp688(depumpPow)\trMOTpow1\tODTpowX(DipPowX)\tfreq\tHeatingAmp\t0\tSine\tDetuning\tsingleFreqDet\tDoppCoolDet-DoppCoolSweep\tdopCoolT*1000\tDetuning\tsingleFreqStirDet\t0\t0\r\narm PIXIS\t\tRamp\t1\t.007\t1\t1\t0\t0\t0\t1\t1\t0\t0\t1\t1\t0\t0\t0\t1\t1\t0\t0\t0\t0\t0\t0\t0\t0\t0\t0\t1\t0\t0\t0\t1\t1\t0\tplus_zman\tminus_zman\tcompensation\trMOTcurrF\trMOTpow1\tcombAmplitude(combWidthF)\trMOTdelta(-(rMOTbroadDetuningF +combWidthF/2))\t0\t1\t1\t0\t0\t0\t1\t1\t1\tbMOTdelta(MOTdetuning)\tbMOTpow(0.5)\tProbePow\tPdet\tXshim\tYshim\tZshimVar\tODTpowZ(DipPowZ)\t1\t0\t0\t0\t0\t0\t0\t0\t0\t0\t0\t0\t0\t0\t0\t0\t0\t0\trMOTdelta(-(rMOTstirDetI +stirWidthF/2))\tcombAmplitude(stirWidthF)\t0\tvarWaveP2\tPdet\tAmp688(depumpPow)\trMOTpow1\tODTpowX(DipPowX)\tfreq\tHeatingAmp\t0\tSine\tDetuning\tsingleFreqDet\tDoppCoolDet-DoppCoolSweep\tdopCoolT*1000\tDetuning\tsingleFreqStirDet\t0\t0\r\narm FLEA\t\tRamp\t1\t44e-6\t1\t1\t0\t0\t0\t1\t1\t0\t0\t1\t1\t0\t0\t0\t1\t1\t0\t0\t0\t0\t0\t0\t0\t0\t0\t0\t1\t0\t0\t0\t1\t0\t0\tplus_zman\tminus_zman\tcompensation\trMOTcurrF\trMOTpow1\tcombAmplitude(combWidthF)\trMOTdelta(-(rMOTbroadDetuningF +combWidthF/2))\t0\t1\t1\t0\t0\t0\t1\t1\t0\tbMOTdelta(MOTdetuning)\tbMOTpow(0.5)\tProbePow\tPdet\tXshim\tYshim\tZshimVar\tODTpowZ(DipPowZ)\t1\t0\t0\t0\t0\t0\t0\t0\t0\t0\t0\t0\t0\t0\t0\t0\t0\t0\trMOTdelta(-(rMOTstirDetI +stirWidthF/2))\tcombAmplitude(stirWidthF)\t0\tvarWaveP2\tPdet\tAmp688(depumpPow)\trMOTpow1\tODTpowX(DipPowX)\tfreq\tHeatingAmp\t0\tSine\tDetuning\tsingleFreqDet\tDoppCoolDet-DoppCoolSweep\tdopCoolT*1000\tDetuning\tsingleFreqStirDet\t0\t0\r\nbg img\t\tRamp\t1\t10e-6\t1\t1\t0\t0\t0\t1\t1\t0\t0\t1\t1\t0\t0\t0\t1\t1\t0\t0\t0\t0\t0\t0\t0\t0\t0\t0\t1\t0\t0\t0\t1\t0\t0\tplus_zman\tminus_zman\tcompensation\trMOTcurrF\trMOTpow1\tcombAmplitude(combWidthF)\trMOTdelta(-(rMOTbroadDetuningF +combWidthF/2))\t0\t1\t1\t0\t0\t0\t1\t0\t0\tbMOTdelta(MOTdetuning)\tbMOTpow(0.5)\tProbePow\tPdet\tXshim\tYshim\tZshimVar\tODTpowZ(DipPowZ)\t1\t0\t0\t0\t0\t0\t0\t0\t0\t0\t0\t0\t0\t0\t0\t0\t0\t0\trMOTdelta(-(rMOTstirDetI +stirWidthF/2))\tcombAmplitude(stirWidthF)\t0\tvarWaveP2\tPdet\tAmp688(depumpPow)\trMOTpow1\tODTpowX(DipPowX)\tfreq\tHeatingAmp\t0\tSine\tDetuning\tsingleFreqDet\tDoppCoolDet-DoppCoolSweep\tdopCoolT*1000\tDetuning\tsingleFreqStirDet\t0\t0\r\nbg img\t\tRamp\t0\t2.8e-3\t1\t1\t0\t0\t0\t1\t1\t0\t0\t1\t1\t0\t0\t0\t1\t1\t0\t0\t0\t0\t0\t0\t0\t0\t0\t0\t1\t0\t0\t0\t1\t1\t0\tplus_zman\tminus_zman\tcompensation\trMOTcurrF\trMOTpow1\tcombAmplitude(combWidthF)\trMOTdelta(-(rMOTbroadDetuningF +combWidthF/2))\t0\t1\t1\t0\t0\t0\t1\t1\t1\tbMOTdelta(MOTdetuning)\tbMOTpow(0.5)\tProbePow\tPdet\tXshim\tYshim\tZshimVar\tODTpowZ(DipPowZ)\t1\t0\t0\t0\t0\t0\t0\t0\t0\t0\t0\t0\t0\t0\t0\t0\t0\t0\trMOTdelta(-(rMOTstirDetI +stirWidthF/2))\tcombAmplitude(stirWidthF)\t0\tvarWaveP2\tPdet\tAmp688(depumpPow)\trMOTpow1\tODTpowX(DipPowX)\tfreq\tHeatingAmp\t0\tSine\tDetuning\tsingleFreqDet\tDoppCoolDet-DoppCoolSweep\tdopCoolT*1000\tDetuning\tsingleFreqStirDet\t0\t0\r\ntransmit img\t\tRamp\t1\t.3\t1\t1\t0\t0\t0\t1\t1\t0\t0\t1\t1\t0\t0\t0\t1\t1\t0\t0\t0\t0\t0\t0\t0\t0\t0\t0\t1\t0\t0\t0\t1\t1\t0\tplus_zman\tminus_zman\tcompensation\trMOTcurrF\trMOTpow1\tcombAmplitude(combWidthF)\trMOTdelta(-(rMOTbroadDetuningF +combWidthF/2))\t0\t1\t1\t0\t0\t0\t1\t1\t1\tbMOTdelta(MOTdetuning)\tbMOTpow(0.5)\tProbePow\tLineRamp(f,Pdet,Pdet2)\tXshim\tYshim\tZshimVar\tODTpowZ(DipPowZ)\t1\t0\t0\t0\t0\t0\t0\t0\t0\t0\t0\t0\t0\t0\t0\t0\t0\t0\trMOTdelta(-(rMOTstirDetI +stirWidthF/2))\tcombAmplitude(stirWidthF)\t0\tvarWaveP2\tPdet\tAmp688(depumpPow)\trMOTpow1\tODTpowX(DipPowX)\tfreq\tHeatingAmp\t0\tSine\tDetuning\tsingleFreqDet\tDoppCoolDet-DoppCoolSweep\tdopCoolT*1000\tDetuning\tsingleFreqStirDet\t0\t0\r\nalignment\t\tRamp\t1\t.5\t1\t1\t0\t0\t1\t1\t1\t0\t0\t0\t1\t0\t1\t1\t1\t1\t0\t0\t0\t0\t0\t0\t0\t0\t1m\t0\t1\t0\t1\t0\t0\t1\t1\tplus_zman\tminus_zman\tcompensation\tMOTcurrent\trMOTpow1\tcombAmplitude(combWidthI)\trMOTdelta(-(rMOTbroadDetuningI +combWidthI/2))\t0\t1\t0\t1\t1\t0\t1\t1\t1\tbMOTdelta(MOTdetuning)\tbMOTpow(MOTPow)\tProbePow\tPdet2\tXshim\tYshim\tZshim\tODTpowZ(DipPowZ)\t0\tdepumpOn\t0\t0\t0\t0\t0\t0\t0\t0\t0\t0\t0\t0\t0\t0\t0\t0\trMOTdelta(-(rMOTstirDetI +stirWidthI/2))\tcombAmplitude(stirWidthI)\t0\tvarWaveP2\tLineRamp(f,Pdet,BlueLaserLockOffset)\tAmp688(depumpPow)\trMOTpow3\tODTpowX(DipPowX2)\tfreq\tHeatingAmp\t0\tSine\tDetuning\tsingleFreqDet\tDoppCoolDet-DoppCoolSweep\tdopCoolT*1000\tDetuning\tsingleFreqStirDet\t0\t0\r\n\r\n\r\n"
  in  "Save files to archive?":bool
  out "Timeout":bool=TRUE
  out "Trigger Overrun":bool=TRUE
  in  "Source of File Data":refnum<k21>="\\\\localhost\\VariableLibrary\\Instruction String"
  in  "Timeout (ms)":u32=1000
  in  "Gain":dbl
  in  "Shutter speed (ms)":dbl=0.15
  in  "Source of Wavemeter Data":refnum<k21>="\\\\WS7PC\\VariableLibrary\\Frequency"
  in  "Accept wavelength from remote system":bool
  in  "AnalysisType":enum16{"AbsGaussFit", "absDipole", "absLineFit"}(ring)
  out "Zoomed in processed image":sgl[][](graph)
  in  "Flea Raw image to view":u16(ring) items=["Absorbtion", "Probe", "Background"]
  in  "Update Graphics":bool=TRUE
  out "Flea Raw Image":u16[][](graph)
  out "Flea Processed Image":sgl[][](graph)
  in  "Height":i32
  in  "Col":i32
  in  "Row":i32
  in  "Width":i32
  out "Camera Error":errorcluster={"status"=FALSE, "code"=-1074360293, "source"="IMAQdx Get Image.vi"}
  out "Status Array":T4(array[cluster])=[{"AcquisitionInProgress"=FALSE, "BufferCount"=1164, "LastBufferNumber"=1163, "LostBufferCount"=0}, {"AcquisitionInProgress"=TRUE, "BufferCount"=12297, "LastBufferNumber"=12296, "LostBufferCount"=0}, {"AcquisitionInProgress"=TRUE, "BufferCount"=12298, "LastBufferNumber"=12297, "LostBufferCount"=0}, {"AcquisitionInProgress"=TRUE, "BufferCount"=12299, "LastBufferNumber"=12298, "LostBufferCount"=0}, {"AcquisitionInProgress"=TRUE, "BufferCount"=12300, "LastBufferNumber"=12299, "LostBufferCount"=0}]